vi "UHR-Fleezers Control (host) - 12.8.vi"() -> ()   [LabVIEW 2012] (continued)
                n1749 = Divide "X pix/step"(x=w2623, y=w2626) -> (x/y=w2632:dbl)
                n1750 = Negate(x=w2635) -> (-x=w2636:dbl)
                n1751 = local read "Initial Y"() -> (w2642:dbl)
                n1752 = Multiply(x=w2624, y=w2633) -> (x*y=w2643:dbl)
                n1753 = Divide "X half step offset"(x=w2621, y=2.0) -> (x/y=w2629:dbl)
                n1754 = Divide "X V/pix"(x=w2621, y=w2632) -> (x/y=w2631:dbl)
                n1755 = Multiply(x=w2621, y=w2626) -> (x*y=w2638:dbl)
                n1756 = Compound Arithmetic op=ADD(w2636, w2643, w2642) -> (w2613:dbl)
                "Pointer Y (V)" <- w2613
                n1757 = Multiply(x=w2631, y=w2625) -> (x*y=w2640:dbl)
                n1758 = Negate(x=w2629) -> (-x=w2628:dbl)
                n1759 = local read "Initial X"() -> (w2641:dbl)
                n1760 = Negate(x=w2640) -> (-x=w2639:dbl)
                n1761 = Compound Arithmetic op=ADD(w2628, w2638, w2641, w2639) -> (w2614:dbl)
                "Pointer X (V)" <- w2614
                n1762 = case shown="True" "Set High F Confocal Spot (X-Y)" {
                  tunnel: w2614 -> [_ w2644]
                  tunnel: w2613 -> [_ w2645]
                  frame False {
                  }
                  frame True {
                    "Confocal Y 2 (V)" <- w2645
                    "Confocal X 2 (V)" <- w2644
                  }
                }
                n1763 = Or(x="Set X Only", y="Set Confocal Spot (X-Y)") -> (x .or. y?=w2617:bool)
                n1764 = Or(x="Set Confocal Spot (X-Y)", y="Set Y Only") -> (x .or. y?=w2616:bool)
                n1765 = case shown="True" w2617 {
                  tunnel: w2614 -> [_ w2646]
                  frame False {
                  }
                  frame True {
                    n1766 = property on="AO2" class="Slide (strict)"("Val(Sgnl)"=w2646) -> ()  [unwired: 2 in, 2 out]
                    "Confocal X 1 (V)" <- w2646
                  }
                }
                n1767 = case shown="True" w2616 {
                  tunnel: w2613 -> [_ w2647]
                  frame False {
                  }
                  frame True {
                    n1768 = property on="AO1" class="Slide (strict)"("Val(Sgnl)"=w2647) -> ()  [unwired: 2 in, 2 out]
                    "Confocal Y 1 (V)" <- w2647
                  }
                }
                n1769 = local write "Set High F Confocal Spot (X-Y)"(w2612) -> ()
                n1770 = local write "Set Confocal Spot (X-Y)"(w2612) -> ()
                n1771 = local write "Set X Only"(w2612) -> ()
                n1772 = local write "Set Y Only"(w2612) -> ()
              }
            }
          }
          frame 3 {
            n1773 = local read "BD 2 Frequency 1 (MHz)"() -> (w2649:dbl)
            n1774 = local read "BD 1 Frequency 1 (MHz)"() -> (w2650:dbl)
            n1775 = local write "Manipulating Trap"(TRUE ("Manipulating Trap")) -> ()
            n1776 = local write "Coords"(T7 {"Horizontal"=0, "Vertical"=0} ("Coords")) -> ()
            n1777 = while {
              tunnel: w2654 -> [w2659]
              tunnel: w2652 -> [w2658]
              tunnel: w2650 -> [w2657]
              tunnel: w2649 -> [w2656]
              tunnel: w2648 -> [w2655]
              stop <- w2660 stop-if-true
              n1778 = event shown="[0] \"Pane\": Mouse Move" {
                selector: _ -> [_ _]
                dyn-events: _ -> [_ _]
                timeout: _ -> [_ _]
                tunnel: ["Force Manip Abort" w2724] -> w2660
                tunnel: w2659 -> [w2667 _]
                tunnel: w2658 -> [w2665 _]
                tunnel: w2657 -> [w2664 _]
                tunnel: w2656 -> [w2663 _]
                tunnel: w2655 -> [w2661 _]
                event Mouse Move {
                  n1779 = event-data() -> ("Time"=w2668:u32, "Coords"=w2669:T7)  [unwired: 3 out]
                  n1780 = Less?(x=w2668, y=w2667) -> (x < y?=w2666:bool)
                  n1781 = case "Makes sure old motion events prior to mouse click aren't used" shown="False" w2666 {
                    tunnel: w2669 -> [w2711 _]
                    tunnel: w2665 -> [w2712 _]
                    tunnel: w2664 -> [w2686 _]
                    tunnel: w2663 -> [w2685 _]
                    tunnel: w2661 -> [w2670 _]
                    frame False {
                      n1782 = Subtract(x=w2711, y=w2712) -> (x-y=w2710:T7)
                      "Coords" <- w2710
                      n1783 = local read "Y RF Frequency Limits (MHz)"() -> (w2671:T16)
                      n1784 = To Double Precision Float(number=w2710) -> (double precision float=w2709:cluster{"Horizontal":dbl, "Vertical":dbl})
                      n1785 = Multiply(x=cluster{"Horizontal":dbl, "Vertical":dbl} {"Horizontal"=-1.0, "Vertical"=1.0}, y="Manipulation Scaling") -> (x*y=w2705:cluster{"Horizontal":dbl, "Vertical":dbl})
                      n1786 = local read "X RF Frequency Limits (MHz)"() -> (w2672:T16)
                      n1787 = Multiply(x=w2709, y=w2705) -> (x*y=w2707:cluster{"Horizontal":dbl, "Vertical":dbl})
                      n1788 = Unbundle By Name(w2707) -> ("Horizontal"=w2702:dbl, "Vertical"=w2706:dbl)
                      n1789 = Unbundle By Name(w2671) -> ("Maximum"=w2674:dbl, "Minimum"=w2673:dbl)
                      n1790 = Boolean To (0,1)(Boolean="Manip. X?") -> (0, 1=w2700:i16)
                      n1791 = Boolean To (0,1)(Boolean="Manip. Y?") -> (0, 1=w2697:i16)
                      n1792 = local read "BD 1 Frequency 2 (MHz)"() -> (w2688:dbl)
                      n1793 = Multiply(x=w2706, y=w2697) -> (x*y=w2699:dbl)
                      n1794 = Multiply(x=w2700, y=w2702) -> (x*y=w2703:dbl)
                      n1795 = local read "BD 2 Frequency 2 (MHz)"() -> (w2687:dbl)
                      n1796 = Unbundle By Name(w2672) -> ("Maximum"=w2676:dbl, "Minimum"=w2675:dbl)
                      n1797 = Add(x=w2685, y=w2699) -> (x+y=w2678:dbl)
                      n1798 = Add(x=w2686, y=w2703) -> (x+y=w2680:dbl)
                      n1799 = In Range and Coerce(upper limit=w2676, x=w2680, lower limit=w2675) -> (coerced(x)=w2679:dbl)  [unwired: 1 out]
                      n1800 = In Range and Coerce(upper limit=w2674, x=w2678, lower limit=w2673) -> (coerced(x)=w2677:dbl)  [unwired: 1 out]
                      n1801 = Subtract(x=w2679, y=w2688) -> (x-y=w2696:dbl)
                      n1802 = Subtract(x=w2677, y=w2687) -> (x-y=w2695:dbl)
                      n1803 = Square(x=w2696) -> (x^2=w2694:dbl)
                      n1804 = Square(x=w2695) -> (x^2=w2693:dbl)
                      n1805 = Add(x=w2694, y=w2693) -> (x+y=w2692:dbl)
                      n1806 = Square Root(x=w2692) -> (sqrt(x)=w2689:dbl)
                      n1807 = In Range and Coerce(upper limit="Limit Max (MHz)", x=w2689, lower limit="Limit Min (MHz)") -> (In Range?=w2682:bool)  [unwired: 1 out]
                      n1808 = Not(x="Limits Enable") -> (.not. x?=w2681:bool)
                      n1809 = Or(x=w2682, y=w2681) -> (x .or. y?=w2683:bool)
                      n1810 = case shown="True" w2683 {
                        tunnel: w2689 -> [_ w2714]
                        tunnel: w2679 -> [_ w2721]
                        tunnel: w2688 -> [_ w2720]
                        tunnel: w2677 -> [_ w2719]
                        tunnel: w2687 -> [_ w2718]
                        tunnel: w2672 -> [_ w2716]
                        tunnel: w2671 -> [_ w2715]
                        tunnel: w2670 -> [_ w2713]
                        frame False {
                        }
                        frame True {
                          n1811 = local read "BD 1 Frequency 3 (MHz)"() -> (w2722:dbl)
                          n1812 = local read "BD 2 Frequency 3 (MHz)"() -> (w2717:dbl)
                          n1813 = local write "Trap Delta (MHz)"(w2714) -> ()
                          n1814 = call "set RF board frequency - interlace.vi"("Board 2 Frequency Limits"=w2715, "Board 1 Frequency Limits"=w2716, "FPGA VI Reference In"=w2713, "Board 2 Frequency 3 (MHz)"=w2717, "Board 1 Frequency 3 (MHz)"=w2722, "Board 2 Frequency 2 (MHz)"=w2718, "Board 2 Frequency 1 (MHz)"=w2719, "Board 1 Frequency 2 (MHz)"=w2720, "Board 1 Frequency 1  (MHz)"=w2721) -> ()  [unwired: 1 in, 2 out]
                          n1815 = local write "BD 2 Frequency 1 (MHz)"(w2719) -> ()
                          n1816 = local write "BD 1 Frequency 1 (MHz)"(w2721) -> ()
                        }
                      }
                    }
                    frame True {
                    }
                  }
                }
                event Mouse Up {
                  n1817 = event-data() -> ("Button"=w2723:u16)  [unwired: 8 out]
                  n1818 = case shown="3" w2723 {
                    tunnel: [FALSE TRUE] -> w2724
                    frame 0, Default {
                    }
                    frame 3 {
                      n1819 = local read "Trap Delta (MHz)"() -> (w2726:dbl)
                      n1820 = property on="Initial delta (MHz)" class="DigNum (strict)"("Val(Sgnl)"=w2726) -> ()  [unwired: 2 in, 2 out]
                      n1821 = local write "Manipulating Trap"(FALSE ("Manipulating Trap")) -> ()
                    }
                  }
                }
              }
            }
          }
        }
      }
      event Mouse Move {
        n1822 = event-data() -> ()  [unwired: 6 out]
      }
    }
    n1823 = local read "Stop All"() -> (w2542:bool)
    n1824 = node-c288() -> ()  [unwired: 2 out]
  }
  n1825 = flat-sequence "Video" {
    tunnel: [w2739] -> w55
    tunnel: w55 -> [w2780]
    frame #0 {
      w2729 = FALSE ("File open?")
      n1826 = while {
        stop <- w2731 continue-if-true
        n1827 = call "Close Video Capture.vi"() -> ("error code OUT"=w2733:i32)
        n1828 = Equal?(x=w2733, y=0) -> (x = y?=w2731:bool)
      }
      n1829 = local write "New Video File"(w2729) -> ()
      n1830 = local write "File open?"(w2729) -> ()
      n1831 = local write "Save Video"(w2729) -> ()
      n1832 = local write "Stop All"(FALSE ("Stop All")) -> ()
    }
    frame #1 {
      n1833 = call "DMR_Init.vi"() -> ()  [unwired: 3 out]
    }
    frame #2 {
      w2734 = "DE245428202"  # MSU fleezers card #
      (unwired) "DE019116701"  # Illinois fleezers card #
      # "Setting the destination format to Mono8 makes sure that the image can be displayed in the intensity plot."
      n1834 = call "DMR_GetDevice.vi"("search string IN"=w2734) -> ("device handle OUT"=w2757:i32)  [unwired: 4 in, 2 out]
      n1835 = call "DMR_OpenDevice.vi"("device handle IN"=w2757) -> ("driver handle OUT"=w2740:i32)  [unwired: 4 out]
      n1836 = call "DMR_FindList.vi"("flags IN"=u32 0 ("flags"), "list name IN"="" ("String"), "list type IN"=T35."camera descriptions", "driver handle IN"=w2740) -> ("list handle OUT"=w2743:i32)  [unwired: 2 out]
      n1837 = call "DMR_FindList.vi"("flags IN"=u32 0 ("flags"), "list name IN"="Base", "list type IN"=T35."setting", "driver handle IN"=w2740) -> ("list handle OUT"=w2741:i32)  [unwired: 2 out]
      n1838 = call "OBJ_GetHandle.vi"("object name IN"="VideoStandard", "list handle IN"=w2743) -> ("object handle OUT"=w2737:i32)  [unwired: 3 out]
      n1839 = call "OBJ_GetHandle.vi"("object name IN"="PixelFormat", "list handle IN"=w2741) -> ("object handle OUT"=w2751:i32)  [unwired: 3 out]
      n1840 = call "OBJ_SetS.vi"("value index IN"=0, "value IN"="NTSC M", "object handle IN"=w2737) -> ()  [unwired: 2 out]
      n1841 = call "OBJ_SetS.vi"("value index IN"=0, "value IN"="Mono8" ("value"), "object handle IN"=w2751) -> ()  [unwired: 2 out]
      n1842 = call "OBJ_GetHandle.vi"("object name IN"="VideoChannel", "list handle IN"=w2741) -> ("object handle OUT"=w2747:i32)  [unwired: 3 out]
      n1843 = while {
        tunnel: [w2761] -> w2739
        tunnel: w2740 -> [w2758]
        stop <- w2759 continue-if-true
        n1844 = call "DMR_ImageRequestSingle.vi"("request control IN"=0, "driver handle IN"=w2758) -> ("error code OUT"=w2760:i32, "driver handle OUT"=w2761:i32)  [unwired: 2 out]
        n1845 = Equal To 0?(x=w2760) -> (x = 0?=w2759:bool)
      }
      n1846 = call "OBJ_SetI.vi"("value index IN"=0, "value IN"=3 ("Video channel"), "object handle IN"=w2747) -> ()  [unwired: 2 out]
    }
    frame #3 {
      w2768 = T19 0 items=["Grayscale (U8)", "Grayscale (I16)", "Grayscale (SGL)", "Complex (CSG)", "RGB (U32)", "HSL (U32)", "RGB (U64)"] ("Image Type")
      w2776 = T19 0 items=["Grayscale (U8)", "Grayscale (I16)", "Grayscale (SGL)", "Complex (CSG)", "RGB (U32)", "HSL (U32)", "RGB (U64)"] ("Image Type")
      n1847 = call "IMAQ AVI2 Get Codec Names"() -> ("Codec Names"=w2763:string[])  [unwired: 10 in, 1 out]
      "Installed Codec Names" <- w2763
      n1848 = for "Create Greyscale map" {
        N: 256 -> [_]
        tunnel: [w2782] -> w2765 mode=indexing
        workers-P: _ -> [_]
        i -> [w2785]
        n1849 = To Unsigned Byte Integer(number=w2785) -> (unsigned 8bit integer=w2781:u8)
        n1850 = Join Numbers(hi=w2781, lo=w2781) -> ((hi.lo)=w2784:u16)
        n1851 = Join Numbers(hi=w2781, lo=w2781) -> ((hi.lo)=w2783:u16)
        n1852 = Join Numbers(hi=w2784, lo=w2783) -> ((hi.lo)=w2782:u32)
      }
      n1853 = property on="Codec choice" class="CmbBox"("Strings[]"=w2763) -> ()  [unwired: 2 in, 2 out]
      n1854 = call "IMAQ Create"("Image Name"="Scaled video", "Image Type"=w2768) -> ("New Image"=w2767:T2)  [unwired: 2 in, 2 out]
      n1855 = call "IMAQ Create"("Image Name"="Main video", "Image Type"=w2776) -> ("New Image"=w2777:T2)  [unwired: 2 in, 2 out]
      n1856 = node-c288(0 ("Processor")) -> (w2775:T23)  [unwired: 3 out]
      n1857 = Initialize Array(u32 0 ("Window Number (0...15)"), 480 ("dimension size"), 640 ("dimension size")) -> (w2770:u32[][])
      n1858 = timed-loop {
        tunnel: w2780 -> [w2802]
        tunnel: [w2801] -> w2779
        tunnel: w2777 -> [w2800]
        timing: w2775 -> [_]
        timing-out: [_] -> w2774
        tunnel: w2770 -> [w2793]
        tunnel: w2767 -> [w2791]
        tunnel: w2765 -> [w2790]
        stop <- w2792 stop-if-true
        # "This block performs the \nactual image capture."
        n1859 = node-c288() -> (→"Finished Late? [i-1]":bool)  [unwired: 5 out]
        n1860 = local read "Stop All"() -> (w2792:bool)
        n1861 = feedback #1(T36 refnum ("AVI Refnum")) -> (w2798:T36)
        n1862 = case shown="True" "New Video File" {
          tunnel: [w2815 w2816] -> w2789
          tunnel: w2798 -> [w2815 w2817]
          frame False {
          }
          frame True {
            n1863 = flat-sequence {
              tunnel: w2817 -> [w2819]
              tunnel: [w2821] -> w2816
              frame #0 {
                n1864 = local read "File open?"() -> (w2818:bool)
                n1865 = case shown="True" w2818 {
                  tunnel: w2819 -> [_ w2820]
                  frame False {
                  }
                  frame True {
                    n1866 = call "IMAQ AVI2 Close"("AVI Refnum"=w2820) -> ()  [unwired: 10 in, 1 out]
                  }
                }
              }
              frame #1 {
                n1867 = local write "New Video File"(FALSE ("New Video File")) -> ()
                n1868 = call "Create new save file.vi"("Ext"=".avi" ("string"), "Index In"="Video Index") -> ("Path Out"=w2824:path, "Index Out"=w2826:dbl)  [unwired: 1 in]
                "Path Out" <- w2824
                n1869 = local write "Video Index"(w2826) -> ()
                n1870 = call "IMAQ AVI2 Create"("Codec"="Codec choice", "Frames Per Second"=u32 30, "AVI Path"=w2824) -> ("AVI Refnum"=w2821:T36)  [unwired: 7 in, 1 out]
                "File open?" <- TRUE ("Files open?")
              }
            }
          }
        }
        n1871 = feedback-in #1(w2789) -> ()
        n1872 = call "DMR_ImageRequestWaitFor.vi"("queue number IN"=0, "timeout(ms) IN"=500, "driver handle IN"=w2802) -> ("error code OUT"=w2806:i32, "request number OUT"=w2803:i32, "driver handle OUT"=w2804:i32)
        n1873 = Equal To 0?(x=w2806) -> (x = 0?=w2805:bool)
        n1874 = Reciprocal(x="Video Capture Rate (Hz)") -> (1/x=w2796:dbl)
        n1875 = Multiply(x=w2796, y=1000.0) -> (x*y=w2794:dbl)
        n1876 = case shown="True" w2805 {
          tunnel: w2804 -> [w2830 w2867]
          tunnel: w2803 -> [_ w2866]
          tunnel: [w2830 w2863] -> w2801
          tunnel: w2800 -> [_ w2849]
          tunnel: w2793 -> [_ w2852]
          tunnel: w2789 -> [_ w2832]
          tunnel: w2791 -> [_ w2846]
          tunnel: w2790 -> [_ w2845]
          frame False {
          }
          frame True {
            w2857 = u32 0 ("X-offset IN")
            n1877 = call "DMR_GetImageRequestBufferData.vi"("driver handle IN"=w2867, "request number IN"=w2866) -> ("width OUT"=w2856:i32, "height OUT"=w2855:i32, "driver handle OUT"=w2862:i32, "request number OUT"=w2861:i32, "bytes per pixel OUT"=w2858:i32)  [unwired: 13 out]
            n1878 = call "DMR_GetImageRequestBufferImageData.vi"("driver handle IN"=w2862, "request number IN"=w2861, "bytes per pixel IN"=w2858, "X-offset IN"=w2857, "Y-offset IN"=w2857, "height IN"=w2855, "width IN"=w2856) -> ("driver handle OUT"=w2860:u32, "request number OUT"=w2859:u32, "image OUT"=w2838:u32[][])  [unwired: 10 out]
            n1879 = Transpose 2D Array(2D array=w2838) -> (transposed array=w2844:u32[][])
            n1880 = Select(t=w2844, s="Flip Y (or X)", f=w2838) -> (s? t:f=w2843:u32[][])
            n1881 = call "DMR_ImageRequestUnlock.vi"("request number IN"=w2859, "driver handle IN"=w2860) -> ("driver handle OUT"=w2865:i32)  [unwired: 1 in, 2 out]
            n1882 = for {
              tunnel: w2843 -> [w2902] mode=indexing
              tunnel: [w2901] -> w2841 mode=indexing
              n1883 = Reverse 1D Array(array=w2902) -> (reversed array=w2901:u32[])
            }
            n1884 = call "DMR_ImageRequestSingle.vi"("request control IN"=0, "driver handle IN"=w2865) -> ("driver handle OUT"=w2863:i32)  [unwired: 3 out]
            n1885 = Transpose 2D Array(2D array=w2841) -> (transposed array=w2842:u32[][])
            n1886 = Select(t=w2842, s="Flip Y (or X)", f=w2841) -> (s? t:f=w2839:u32[][])
            n1887 = Select(t=w2839, s="Flip Image", f=w2838) -> (s? t:f=w2836:u32[][])
            n1888 = case shown="True" "Averaging" {
              tunnel: w2836 -> [w2913 w2918]
              tunnel: [w2913 w2917] -> w2850
              tunnel: w2852 -> [_ w2915]
              frame False {
              }
              frame True {
                (unwired) 1
                w2923 = 1
                n1889 = feedback #2(w2915) -> (w2914:u32[][])
                n1890 = Add(x=w2918, y=w2914) -> (x+y=w2919:u32[][])
                n1891 = Select(t=w2915, s="Reset Averaging", f=w2919) -> (s? t:f=w2921:u32[][])
                n1892 = feedback-in #2(w2921) -> ()
                n1893 = feedback #3(w2923) -> (w2916:i32)
                n1894 = Divide(x=w2919, y=w2916) -> (x/y=w2920:dbl[][])
                n1895 = Increment(x=w2916) -> (x+1=w2924:i32)
                n1896 = To Unsigned Long Integer(number=w2920) -> (unsigned 32bit integer=w2917:u32[][])
                n1897 = Select(t=w2923, s="Reset Averaging", f=w2924) -> (s? t:f=w2922:i32)
                n1898 = feedback-in #3(w2922) -> ()
              }
            }
            n1899 = case shown="True" "Zoom video window" {
              tunnel: w2850 -> [_ w2881]
              tunnel: w2846 -> [_ w2880]
              frame False {
              }
              frame True {
                n1900 = To Double Precision Float(number=w2881) -> (double precision float=w2878:dbl[][])
                n1901 = In Range and Coerce(upper limit="Intensity Upper", x=w2878, lower limit="Intensity Lower") -> (coerced(x)=w2877:dbl[][])  [unwired: 1 out]
                n1902 = Subtract(x="Intensity Upper", y="Intensity Lower") -> (x-y=w2874:dbl)
                n1903 = Subtract(x=w2877, y="Intensity Lower") -> (x-y=w2875:dbl[][])
                n1904 = Divide(x=w2875, y=w2874) -> (x/y=w2876:dbl[][])
                n1905 = Multiply(x=255.0, y=w2876) -> (x*y=w2872:dbl[][])
                n1906 = To Unsigned Byte Integer(number=w2872) -> (unsigned 8bit integer=w2879:u8[][])
                n1907 = call "IMAQ ArrayToImage"("Image Pixels (U8)"=w2879, "Image"=w2880) -> ("Image Out"=w2868:T2)  [unwired: 4 in, 5 out]
                n1908 = First Call?() -> (First Call?: T/F=w2869:bool)
                n1909 = case shown="True" w2869 {
                  tunnel: w2868 -> [w2882 w2893]
                  frame False {
                    n1910 = flat-sequence {
                      tunnel: w2882 -> [w2888]
                      frame #0 {
                        w2885 = FALSE ("Get/Set Status? (Set)")
                        w2884 = 0 ("Window Number (0...15)")
                        n1911 = call "IMAQ WindSize"("Get/Set Status? (Set)"=w2885, "Window Number"=w2884) -> ("Width & Height out"=→"Window Size":cluster{"Width":i32, "Height":i32})  [unwired: 4 in, 2 out]
                        n1912 = call "IMAQ WindMove"("Window Number (0...15)"=w2884, "Get/Set Status? (Set)"=w2885) -> ("Coordinates (screen)"=→"Window Position":cluster{"X Position":i32, "Y Position":i32})  [unwired: 3 in, 1 out]
                        n1913 = call "IMAQ WindDraw"("Resize to Image Size? (Y)"=FALSE, "Window Number (0...15)"=w2884, "Image"=w2888) -> ()  [unwired: 7 in, 2 out]
                      }
                      frame #1 {
                        n1914 = call "IMAQ WindZoom 2"("Center Point"="Center Point", "Zoom to Fit? (False)"=FALSE, "Zoom Factor"="Zoom Factor") -> ()  [unwired: 5 in, 4 out]
                      }
                    }
                  }
                  frame True {
                    n1915 = flat-sequence {
                      tunnel: w2893 -> [w2896]
                      tunnel: [w2894] -> w2892
                      tunnel: w2892 -> [w2898]
                      frame #0 {
                        w2895 = TRUE ("Resize to Image Size? (Y)")
                        w2894 = 0 ("Window Number (0...15)")
                        n1916 = call "IMAQ WindNonTearing"("Window Number"=w2894, "NonTearing? (True)"=w2895) -> ()  [unwired: 8 in, 2 out]
                        n1917 = call "IMAQ WindDraw"("Resize to Image Size? (Y)"=w2895, "Window Number (0...15)"=w2894, "Image"=w2896) -> ()  [unwired: 7 in, 2 out]
                      }
                      frame #1 {
                        n1918 = call "IMAQ WindSize"("Scrollbars? (N)"=FALSE, "Width & Height"="Initial Window Size", "Window Number"=w2898) -> ()  [unwired: 3 in, 3 out]
                        n1919 = call "IMAQ WindMove"("Window Number (0...15)"=w2898, "Coordinates (screen)"="Initial Window Position") -> ()  [unwired: 3 in, 2 out]
                      }
                    }
                  }
                }
              }
            }
            n1920 = To Unsigned Byte Integer(number=w2850) -> (unsigned 8bit integer=w2848:u8[][])
            n1921 = call "IMAQ ArrayToImage"("Image Pixels (U8)"=w2848, "Image"=w2849) -> ("Image Out"=w2847:T2)  [unwired: 4 in, 5 out]
            "Primary Video Display" <- w2847
            n1922 = Not(x="Close Video File") -> (.not. x?=w2834:bool)
            n1923 = And(x="Save Video", y=w2834) -> (x .and. y?=w2831:bool)
            n1924 = case shown="True" "Save Image" {
              tunnel: w2848 -> [_ w2927]
              tunnel: w2845 -> [_ w2926]
              frame False {
              }
              frame True {
                n1925 = call <vilib>:"Flatten Pixmap.vi"("colors"=w2926, "8-bit pixmap"=w2927) -> ("image data"=w2933:T37)  [unwired: 4 in, 5 out]
                n1926 = call "Create new save file.vi"("Insert"="video_frame_" ("string"), "Ext"=".bmp" ("string"), "Index In"="Image Index") -> ("Path Out"=w2929:path, "Index Out"=w2934:dbl)
                n1927 = Increment(x=w2934) -> (x+1=w2928:dbl)
                n1928 = local write "Image Index"(w2928) -> ()
                n1929 = call <vilib>:"Write BMP File.vi"("image data"=w2933, "path to BMP file"=w2929) -> ()  [unwired: 1 in, 9 out]
              }
            }
            n1930 = case shown="True" w2831 {
              tunnel: w2832 -> [w2904 w2909]
              tunnel: w2847 -> [_ w2908]
              tunnel: "Close Video File" -> [w2903 _]
              frame False {
                n1931 = case shown="True" w2903 {
                  tunnel: w2904 -> [_ w2905]
                  frame False {
                  }
                  frame True {
                    w2906 = FALSE ("Save Video")
                    n1932 = call "IMAQ AVI2 Close"("AVI Refnum"=w2905) -> ()  [unwired: 10 in, 1 out]
                    n1933 = local write "File open?"(w2906) -> ()
                    n1934 = local write "Save Video"(w2906) -> ()
                  }
                }
              }
              frame True {
                n1935 = local read "File open?"() -> (w2907:bool)
                n1936 = case shown="True" w2907 {
                  tunnel: w2909 -> [_ w2912]
                  tunnel: w2908 -> [_ w2911]
                  frame False {
                    n1937 = local write "New Video File"(TRUE ("New Video File")) -> ()
                  }
                  frame True {
                    n1938 = call "IMAQ AVI2 Write Frame"("Image"=w2911, "AVI Refnum"=w2912) -> ()  [unwired: 7 in, 3 out]
                  }
                }
              }
            }
          }
        }
        n1939 = node-c288(w2794, "Deadline (ms)") -> ()  [unwired: 1 out]
      }
      n1940 = node-c288(w2774) -> ()  [unwired: 1 out]
      n1941 = call "DMR_CloseDevice.vi"("driver handle IN"=w2779) -> ()  [unwired: 1 in, 4 out]
    }
    frame #4 {
      n1942 = call "DMR_Close.vi"() -> ()  [unwired: 1 out]
    }
  }
  n1943 = node-c288(3 ("Processor")) -> (w64:T23)  [unwired: 3 out]
  n1944 = timed-loop "Oscillate Trap/AOM (fishing, conjugate plane alignment)" {
    tunnel: [w2940] -> w69
    timing: w64 -> [_]
    timing-out: [_] -> w63
    tunnel: w5 -> [w2939]
    stop <- w2940 stop-if-true
    n1945 = node-c288() -> ()  [unwired: 2 out]
    n1946 = event shown="[0] \"Oscillate Set 1\", \"Fish for Tether\": Value Change" {
      selector: _ -> [_ _ _]
      dyn-events: _ -> [_ _ _]
      timeout: _ -> [_ _ _]
      tunnel: [FALSE ("Stop All") _ w3545] -> w2940
      tunnel: w2939 -> [w2943 _ _]
      event "Oscillate Set 1", "Fish for Tether": Value Change {
        n1947 = event-data() -> ()  [unwired: 6 out]
        n1948 = local read "Oscillate Set 1"() -> (w2947:bool)
        n1949 = Or(x=w2947, y="Fish for Tether") -> (x .or. y?=w2945:bool)
        n1950 = case shown="True" w2945 {
          tunnel: "Fish for Tether" -> [_ w2950]
          tunnel: w2943 -> [_ w2948]
          frame False {
          }
          frame True {
            n1951 = case shown="True" w2950 {
              selector: w2950 -> [w2953 w2959]
              tunnel: [w2953 w2959] -> w2949
              frame False {
              }
              frame True {
                n1952 = local write "Scan axis 2"(TRUE) -> ()
                n1953 = local write "Tether"(FALSE ("Tether")) -> ()
                n1954 = local read "Flow ON during cal?"() -> (w2954:bool)
                n1955 = property on="Trap Delta (MHz)" class="DigNum (strict)"("Val(Sgnl)"="Furthest Delta (MHz)") -> ()  [unwired: 2 in, 2 out]
                n1956 = Or(x="Flow ON during \nfishing?", y=w2954) -> (x .or. y?=w2955:bool)
                n1957 = Wait (ms)(milliseconds to wait=u32 500) -> ()  [unwired: 1 out]
                n1958 = property on="Sample Channel\nFlow" class="Bool (strict)"("Val(Sgnl)"=w2955) -> ()  [unwired: 2 in, 2 out]
              }
            }
            n1959 = node-c288() -> (w2952:T23)  [unwired: 1 in, 3 out]
            n1960 = timed-loop "Oscillate AOD" {
              timing: w2952 -> [_]
              timing-out: [_] -> w2951
              tunnel: w2949 -> [w2963]
              tunnel: w2948 -> [w2962]
              i -> [w2971]
              stop <- w2969 stop-if-true
              n1961 = node-c288() -> (w2970:i64)  [unwired: 1 out]
              n1962 = flat-sequence {
                tunnel: w2971 -> [w2998]
                tunnel: w2970 -> [w2997]
                tunnel: w2963 -> [w2981]
                tunnel: [w2981] -> w2968
                tunnel: [w2980] -> w2967
                tunnel: [w2979] -> w2966
                tunnel: [w2976] -> w2964
                tunnel: w2962 -> [w2972]
                tunnel: w2968 -> [w3043]
                tunnel: w2967 -> [w3041]
                tunnel: w2966 -> [w3040]
                tunnel: [w3039] -> w2965
                tunnel: w2964 -> [w3038]
                tunnel: [w3115] -> w2969
                tunnel: w2965 -> [w3114]
                frame #0 {
                  # "w (rad/s)"
                  # "t (s)"
                  n1963 = Divide(x=w2997, y=i64 1000) -> (x/y=w2973:dbl)
                  n1964 = local read "BD 1 Frequency 2 (MHz)"() -> (w2975:dbl)
                  n1965 = Multiply(x="Osc. freq. (Hz)", y=6.283185307179586) -> (x*y=w2995:dbl)
                  n1966 = Multiply(x=w2973, y=w2998) -> (x*y=w2994:dbl)
                  n1967 = Multiply(x=w2995, y=w2994) -> (x*y=w2978:dbl)
                  n1968 = local read "BD 1 Frequency 1 (MHz)"() -> (w2983:dbl)
                  n1969 = case shown="True" w2981 {
                    tunnel: w2978 -> [w3004 w3021]
                    tunnel: w2983 -> [_ w3029]
                    tunnel: w2975 -> [_ w3030]
                    tunnel: [w3001 w3025] -> w2974
                    tunnel: [FALSE w3006] -> w2979
                    tunnel: [0.0 w3017] -> w2976
                    frame False {
                      n1970 = Sine(x=w3004) -> (sin(x)=w3002:dbl)
                      n1971 = Multiply(x=w3002, y="Osc. amp. (MHz)") -> (x*y=w3001:dbl)
                    }
                    frame True {
                      # "trap position goes from 0 to 1 (0 is when it is furthest away, 1 is when closest)\nso we want to test for tether only when farther away, or x < 1"
                      # "quit if taking too long"
                      # "oscillate the trap"
                      # "Test for tether"
                      n1972 = local read "Vec Mean of T1 T2"() -> (w3005:dbl[])
                      "Trigger Signal" <- w3005
                      n1973 = Cosine(x=w3021) -> (cos(x)=w3033:dbl)
                      n1974 = Subtract(x=w3030, y=w3029) -> (x-y=w3028:dbl)
                      n1975 = Decrement(x=w3033) -> (x-1=w3032:dbl)
                      n1976 = Subtract(x=w3028, y="Closest Delta (MHz)") -> (x-y=w3026:dbl)
                      n1977 = Divide(x=w3032, y=-2.0) -> (x/y=w3016:dbl)
                      n1978 = Greater?(x=w3005, y="Stop F (pN)") -> (0:w3023:bool[])
                      n1979 = Multiply(x=w3016, y=w3026) -> (x*y=w3025:dbl)
                      n1980 = Less?(x=w3016, y="Fish mask thresh") -> (x < y?=w3015:bool)
                      n1981 = Boolean To (0,1)(Boolean=w3015) -> (0, 1=w3013:i16)
                      n1982 = Multiply(x=w3013, y=w3005) -> (x*y=w3012:dbl[])
                      n1983 = Divide(x=w3021, y=6.283185307179586) -> (x/y=w3020:dbl)
                      n1984 = Round Toward +Infinity(x=w3020) -> (ceil(x): smallest int >= x=w3017:dbl)
                      "Attempts" <- w3017
                      n1985 = Greater?(x=w3012, y="Stop F (pN) (mask)") -> (0:w3010:bool[])
                      n1986 = Or Array Elements(Boolean array=w3023) -> (logical OR=w3008:bool)
                      n1987 = Or Array Elements(Boolean array=w3010) -> (logical OR=w3007:bool)
                      n1988 = Greater?(x=w3017, y="Attempt Limit") -> (0:w3019:bool)
                      n1989 = case shown="True" w3019 {
                        frame False {
                        }
                        frame True {
                          n1990 = local write "Fish for Tether"(FALSE ("Fish for Tether")) -> ()
                          n1991 = call <vilib>:"Beep.vi"() -> ()  [unwired: 3 in, 9 out]
                          n1992 = local read "Messages"() -> (w3035:string)
                          n1993 = call "Update messages.vi"("Message to add"="Tether fishing timeout." ("Messages"), "Old message string"=w3035) -> ("New message string"=→"Messages":string)
                        }
                      }
                      n1994 = Select(t=w3008, s="Normal (on) or masked test (off)", f=w3007) -> (s? t:f=w3006:bool)
                    }
                  }
                  n1995 = local read "BD 2 Frequency 1 (MHz)"() -> (w2982:dbl)
                  n1996 = Select(t=w2983, s="Scan axis 2", f=w2982) -> (s? t:f=w2986:dbl)
                  n1997 = Add(x=w2974, y=w2986) -> (x+y=w2980:dbl)
                  n1998 = Select(t=w2980, s="Scan axis 2", f=w2983) -> (s? t:f=w2989:dbl)
                  n1999 = Select(t=w2982, s="Scan axis 2", f=w2980) -> (s? t:f=w2988:dbl)
                  n2000 = local read "BD 2 Frequency 2 (MHz)"() -> (w2991:dbl)
                  n2001 = local read "BD 2 Frequency 3 (MHz)"() -> (w2990:dbl)
                  n2002 = local read "Y RF Frequency Limits (MHz)"() -> (w2984:T16)
                  n2003 = local read "X RF Frequency Limits (MHz)"() -> (w2985:T16)
                  n2004 = local read "BD 1 Frequency 3 (MHz)"() -> (w2992:dbl)
                  n2005 = call "set RF board frequency - interlace.vi"("Board 2 Frequency Limits"=w2984, "Board 1 Frequency Limits"=w2985, "FPGA VI Reference In"=w2972, "Board 2 Frequency 3 (MHz)"=w2990, "Board 1 Frequency 3 (MHz)"=w2992, "Board 2 Frequency 2 (MHz)"=w2991, "Board 2 Frequency 1 (MHz)"=w2988, "Board 1 Frequency 2 (MHz)"=w2975, "Board 1 Frequency 1  (MHz)"=w2989) -> ()  [unwired: 1 in, 2 out]
                }
                frame #1 {
                  n2006 = And(x=w3043, y=w3040) -> (x .and. y?=w3042:bool)
                  n2007 = case "Only if were fishing and now formed tether" shown="True" w3042 {
                    tunnel: w3041 -> [w3045 w3060]
                    tunnel: [w3044 w3059] -> w3039
                    tunnel: w3038 -> [_ w3055]
                    frame False {
                      n2008 = local read "Fish for Tether"() -> (w3044:bool)
                      n2009 = case shown="False" w3044 {
                        tunnel: w3045 -> [w3046 _]
                        frame False {
                          n2010 = property on="BD 1 Frequency 1 (MHz)" class="DigNum (strict)"("Val(Sgnl)"=w3046) -> ()  [unwired: 2 in, 2 out]
                        }
                        frame True {
                        }
                      }
                    }
                    frame True {
                      w3059 = FALSE ("Fish for Tether")
                      n2011 = call <vilib>:"Beep.vi"() -> ()  [unwired: 3 in, 9 out]
                      n2012 = Number To Decimal String(number=w3055, width (-)=i16 1) -> (decimal integer string=w3053:string)
                      n2013 = Concatenate Strings("Formed tether in ", w3053, " attempt(s)." ("string")) -> (w3050:string)
                      n2014 = local read "Messages"() -> (w3057:string)
                      n2015 = local write "Fish for Tether"(w3059) -> ()
                      n2016 = call "Update messages.vi"("Message to add"=w3050, "Old message string"=w3057) -> ("New message string"=w3056:string)
                      n2017 = local write "Messages"(w3056) -> ()
                      n2018 = Get Date/Time In Seconds() -> (seconds since 1Jan1904=→"Time tether formed":timestamp)
                      n2019 = local read "Flow ON during cal?"() -> (w3047:bool)
                      n2020 = property on="Sample Channel\nFlow" class="Bool (strict)"("Val(Sgnl)"=w3047) -> (error out=w3048:errorcluster)  [unwired: 2 in, 1 out]
                      n2021 = case shown="\"2\", \"3\", \"4\", \"5\", \"6\"" "Then..." {
                        selector: "Then..." -> [_ w3063]
                        tunnel: w3060 -> [w3062 _]
                        tunnel: w3048 -> [_ _]
                        frame "1", Default {
                          n2022 = property on="BD 1 Frequency 1 (MHz)" class="DigNum (strict)"("Val(Sgnl)"=w3062) -> ()  [unwired: 2 in, 2 out]
                        }
                        frame "2", "3", "4", "5", "6" {
                          n2023 = flat-sequence {
                            tunnel: w3063 -> [w3065]
                            frame #0 {
                              n2024 = property on="Trap Delta (MHz)" class="DigNum (strict)"("Val(Sgnl)"="Move to Delta 1 (MHz)") -> ()  [unwired: 2 in, 2 out]
                            }
                            frame #1 {
                              n2025 = case shown="\"5\", \"6\"" w3065 {
                                selector: w3065 -> [w3068 w3078 _]
                                frame "3", "4" {
                                n2026 = flat-sequence {
                                tunnel: w3068 -> [w3069]
                                tunnel: [w3069] -> w3066
                                tunnel: [w3071] -> w3067
                                tunnel: w3066 -> [w3071]
                                tunnel: w3067 -> [w3075]
                                frame #0 {
                                n2027 = property on="Green Laser ON" class="Bool (strict)"("Val(Sgnl)"=TRUE ("Value (Signaling)")) -> ()  [unwired: 2 in, 2 out]
                                }
                                frame #1 {
                                n2028 = Multiply(x="Wait Before Save (s)", y=u32 1000 ("x")) -> (x*y=w3073:u32)
                                n2029 = Wait (ms)(milliseconds to wait=w3073) -> ()  [unwired: 1 out]
                                }
                                frame #2 {
                                n2030 = property on="Start Saving" class="Bool (strict)"("Value"=TRUE ("Start Saving")) -> ()  [unwired: 2 in, 2 out]
                                n2031 = case shown="\"4\"" w3075 {
                                frame Default {
                                }
                                frame "4" {
                                n2032 = property on="Fl. Triggered..." class="Bool (strict)"("Val(Sgnl)"=TRUE ("Value (Signaling)")) -> ()  [unwired: 2 in, 2 out]
                                }
                                }
                                }
                                }
                                }
                                frame "5", "6" {
                                n2033 = stacked-sequence {
                                tunnel: w3078 -> [_ _ _ _ _ _ w3090]
                                frame #0 {
                                n2034 = Replace Array Subset(array=u32[] [0] ("Index Values"), new element="Raster Set Upon Tether", index=0) -> (w3079:u32[])
                                n2035 = property on="Saved AOD Raster Scan Parameter Sets" class="Arr (strict)"("Index Values"=w3079) -> ()  [unwired: 2 in, 2 out]
                                }
                                frame #1 {
                                n2036 = Wait (ms)(milliseconds to wait=u32 500) -> ()  [unwired: 1 out]
                                }
                                frame #2 {
                                n2037 = property on="Load parameters" class="Bool (strict)"("Val(Sgnl)"=TRUE ("Value (Signaling)")) -> ()  [unwired: 2 in, 2 out]
                                n2038 = case shown="True" "Green ON During Raster" {
                                frame False {
                                }
                                frame True {
                                n2039 = property on="Green Laser ON" class="Bool (strict)"("Val(Sgnl)"=TRUE ("Value (Signaling)")) -> ()  [unwired: 2 in, 2 out]
                                }
                                }
                                }
                                frame #3 {
                                n2040 = Wait (ms)(milliseconds to wait=u32 500) -> ()  [unwired: 1 out]
                                }
                                frame #4 {
                                n2041 = property on="Trap Raster Scan" class="Bool (strict)"("Val(Sgnl)"=TRUE ("Value (Signaling)")) -> ()  [unwired: 2 in, 2 out]
                                }
                                frame #5 {
                                n2042 = Wait (ms)(milliseconds to wait=u32 2000) -> ()  [unwired: 1 out]
                                }
                                frame #6 {
                                n2043 = flat-sequence {
                                tunnel: w3090 -> [w3097]
                                frame #0 {
                                n2044 = while {
                                stop <- w3093 stop-if-true
                                n2045 = local read "Raster Scanning..."() -> (w3092:bool)
                                n2046 = local read "Saving..."() -> (w3095:bool)
                                n2047 = Wait (ms)(milliseconds to wait=u32 100) -> ()  [unwired: 1 out]
                                n2048 = Not(x=w3095) -> (.not. x?=w3094:bool)
                                n2049 = Not(x=w3092) -> (.not. x?=w3091:bool)
                                n2050 = And(x=w3094, y=w3091) -> (x .and. y?=w3093:bool)
                                }
                                }
                                frame #1 {
                                n2051 = local read "Tether"() -> (w3098:bool)
                                n2052 = case shown="True" w3098 {
                                tunnel: w3097 -> [_ w3100]
                                frame False {
                                n2053 = property on="Fish for Tether" class="Bool (strict)"("Val(Sgnl)"="Fish again after \nraster break?") -> ()  [unwired: 2 in, 2 out]
                                }
                                frame True {
                                n2054 = stacked-sequence {
                                tunnel: w3100 -> [_ w3104 _ _]
                                frame #0 {
                                n2055 = property on="Trap Delta (MHz)" class="DigNum (strict)"("Val(Sgnl)"="Move to Delta 2 (MHz)") -> ()  [unwired: 2 in, 2 out]
                                n2056 = case shown="True" "Flow ON after\ntether testing?" {
                                frame False {
                                }
                                frame True {
                                n2057 = property on="Sample Channel\nFlow" class="Bool (strict)"("Val(Sgnl)"=TRUE ("Value (Signaling)")) -> ()  [unwired: 2 in, 2 out]
                                }
                                }
                                }
                                frame #1 {
                                n2058 = flat-sequence {
                                tunnel: w3104 -> [w3106]
                                frame #0 {
                                n2059 = Wait (ms)(milliseconds to wait=u32 500) -> ()  [unwired: 1 out]
                                }
                                frame #1 {
                                n2060 = case shown="\"6\"" w3106 {
                                frame Default {
                                }
                                frame "6" {
                                n2061 = property on="Green Laser ON" class="Bool (strict)"("Val(Sgnl)"=TRUE ("Green Laser ON/Interlacing")) -> ()  [unwired: 2 in, 2 out]
                                }
                                }
                                }
                                frame #2 {
                                n2062 = Wait (ms)(milliseconds to wait=u32 500) -> ()  [unwired: 1 out]
                                }
                                frame #3 {
                                n2063 = local write "Start Saving"("Save at end (5, 6)") -> ()
                                }
                                }
                                }
                                frame #2 {
                                n2064 = local read "Bead Sep. Int. Time (s)"() -> (w3112:dbl)
                                n2065 = Multiply(x=w3112, y=1000.0) -> (x*y=w3111:dbl)
                                n2066 = Wait (ms)(milliseconds to wait=w3111) -> ()  [unwired: 1 out]
                                }
                                frame #3 {
                                n2067 = property on="Remove Offset" class="Bool (strict)"("Val(Sgnl)"=TRUE ("Value (Signaling)")) -> ()  [unwired: 2 in, 2 out]
                                }
                                }
                                }
                                }
                                }
                                }
                                }
                                }
                                }
                                frame "2", Default {
                                }
                              }
                            }
                          }
                        }
                      }
                      "Tether" <- "Tether Alarm?"
                    }
                  }
                }
                frame #2 {
                  n2068 = local read "Oscillate Set 1"() -> (w3119:bool)
                  n2069 = local read "Stop All"() -> (w3117:bool)
                  n2070 = Or(x=w3119, y=w3114) -> (x .or. y?=w3116:bool)
                  n2071 = Not(x=w3116) -> (.not. x?=w3118:bool)
                  n2072 = Compound Arithmetic op=OR(w3117, w3118) -> (w3115:bool)
                }
              }
              n2073 = node-c288() -> ()  [unwired: 2 out]
            }
            n2074 = node-c288(w2951) -> ()  [unwired: 1 out]
          }
        }
      }
      event "Fl. Triggered...": Value Change {
        n2075 = event-data() -> ()  [unwired: 7 out]
        n2076 = case shown="True" "Fl. Triggered..." {
          frame False {
          }
          frame True {
            n2077 = node-c288() -> (w3130:T23)  [unwired: 4 out]
            n2078 = timed-loop {
              timing: w3130 -> [_]
              timing-out: [_] -> w3129
              tunnel: "Action" -> [w3138]
              shift-right: [w3135] -> _
              shift-left: u8 255 -> [w3137]
              shift-right: [w3132] -> _
              shift-left: 255 -> [w3134]
              stop <- w3131 stop-if-true
              # "Reset confocal spot"
              n2079 = node-c288() -> ()  [unwired: 2 out]
              n2080 = flat-sequence {
                tunnel: w3138 -> [w3158]
                tunnel: w3137 -> [w3157]
                tunnel: [w3156] -> w3136
                tunnel: w3134 -> [w3143]
                tunnel: [w3142] -> w3133
                tunnel: [w3537] -> w3131
                tunnel: w3136 -> [w3536]
                tunnel: [w3536] -> w3135
                tunnel: [w3535] -> w3132
                tunnel: w3133 -> [w3535]
                frame #0 {
                  n2081 = local read "Delta Fl. 2"() -> (w3155:dbl)
                  n2082 = local read "Delta Fl. 1"() -> (w3150:dbl)
                  n2083 = Multiply(x="Fl. Delta Thresh. (kHz)", y=1000.0) -> (x*y=w3145:dbl)
                  n2084 = Select(t=w3150, s="APD to Watch", f=w3155) -> (s? t:f=w3146:dbl)
                  n2085 = Greater?(x=w3146, y=w3145) -> (0:w3151:bool)
                  n2086 = Or(x="Force Yank", y=w3151) -> (x .or. y?=w3149:bool)
                  n2087 = And(x=w3149, y="Yank when?") -> (x .and. y?=w3147:bool)
                  n2088 = case shown="False" w3147 {
                    tunnel: w3158 -> [w3161 w3362]
                    tunnel: w3157 -> [w3163 w3358]
                    tunnel: [w3163 w3356] -> w3156
                    tunnel: w3146 -> [w3169 _]
                    tunnel: w3145 -> [w3168 _]
                    tunnel: "Force Yank" -> [w3166 _]
                    tunnel: w3143 -> [w3165 w3355]
                    tunnel: [w3164 w3355] -> w3142
                    frame False {
                      n2089 = Negate(x=w3168) -> (-x=w3160:dbl)
                      n2090 = local write "Fl. High"(TRUE ("Fl. High")) -> ()
                      n2091 = Less?(x=w3169, y=w3160) -> (x < y?=w3167:bool)
                      n2092 = Or(x=w3166, y=w3167) -> (x .or. y?=w3162:bool)
                      n2093 = case shown="True" w3162 {
                        tunnel: w3165 -> [w3170 w3180]
                        tunnel: [w3170 w3179] -> w3164
                        tunnel: w3161 -> [_ w3178]
                        frame False {
                        }
                        frame True {
                          n2094 = flat-sequence {
                            tunnel: w3180 -> [w3186]
                            tunnel: w3178 -> [w3183]
                            tunnel: [w3185] -> w3177
                            tunnel: [w3184] -> w3176
                            tunnel: [w3183] -> w3175
                            tunnel: w3174 -> [w3182]
                            tunnel: [w3182] -> w3173
                            tunnel: w3172 -> [w3181]
                            tunnel: [w3181] -> w3171
                            tunnel: [w3257] -> w3179
                            tunnel: w3177 -> [w3257]
                            tunnel: w3176 -> [w3256]
                            tunnel: w3175 -> [w3255]
                            tunnel: w3173 -> [w3254]
                            tunnel: w3171 -> [w3253]
                            frame #0 {
                              n2095 = call <vilib>:"Beep.vi"() -> ()  [unwired: 12 in]
                              n2096 = local write "Waiting"(FALSE ("Waiting")) -> ()
                              n2097 = Increment(x=w3186) -> (x+1=w3185:i32)
                              n2098 = case shown="\"Image\"" w3183 {
                                tunnel: w3185 -> [_ w3191 _]
                                frame "Alarm", Default {
                                }
                                frame "Yank" {
                                n2099 = flat-sequence {
                                tunnel: w3191 -> [w3194]
                                tunnel: [w3193] -> w3190
                                tunnel: [w3192] -> w3189
                                tunnel: w3190 -> [w3204]
                                tunnel: w3189 -> [w3205]
                                frame #0 {
                                n2100 = local read "Yank Delay (s)"() -> (w3197:dbl)
                                n2101 = local read "N Array El"() -> (w3192:u8)
                                n2102 = Quotient & Remainder(x=w3194, y=w3192) -> (x-y*floor(x/y)=w3193:i32)  [unwired: 1 out]
                                n2103 = Multiply(x=w3197, y=1000.0) -> (x*y=w3195:dbl)
                                n2104 = Wait (ms)(milliseconds to wait=w3195) -> ()  [unwired: 1 out]
                                }
                                frame #1 {
                                n2105 = local read "Yank to which?"() -> (w3199:bool)
                                n2106 = local read "Random Choice"() -> (w3209:bool)
                                n2107 = local read "Yank to Trap Delta (MHz)"() -> (w3202:dbl[])
                                n2108 = local read "Yank to SP"() -> (w3203:dbl[])
                                n2109 = Random Number (0-1)() -> (number: 0 to 1=w3208:dbl)
                                n2110 = Multiply(x=w3205, y=w3208) -> (x*y=w3207:dbl)
                                n2111 = Round Toward -Infinity(1:w3207) -> (0:w3206:dbl)
                                n2112 = Select(t=w3206, s=w3209, f=w3204) -> (s? t:f=w3200:dbl)
                                n2113 = Select(t=w3202, s=w3199, f=w3203) -> (s? t:f=w3201:dbl[])
                                n2114 = Index Array(array=w3201, index=w3200) -> (element=w3198:dbl)
                                n2115 = case shown="True" w3199 {
                                tunnel: w3198 -> [w3210 w3237]
                                frame False {
                                n2116 = flat-sequence {
                                tunnel: w3210 -> [w3211]
                                frame #0 {
                                n2117 = property on="Trap Pos FB SP" class="DigNum (strict)"("Val(Sgnl)"=w3211) -> ()  [unwired: 2 in, 2 out]
                                }
                                frame #1 {
                                n2118 = Wait (ms)(milliseconds to wait=u32 700) -> ()  [unwired: 1 out]
                                }
                                frame #2 {
                                n2119 = local read "Action (%)"() -> (w3216:dbl)
                                n2120 = Absolute Value(x=w3216) -> (abs(x)=w3215:dbl)
                                n2121 = Greater?(x=w3215, y=70.0) -> (0:w3213:bool)
                                n2122 = property on="Remove Action Offset" class="Bool (strict)"("Val(Sgnl)"=w3213) -> ()  [unwired: 2 in, 2 out]
                                }
                                frame #3 {
                                n2123 = for {
                                N: 4 -> [_]
                                n2124 = flat-sequence {
                                frame #0 {
                                n2125 = Wait (ms)(milliseconds to wait=u32 500) -> ()  [unwired: 1 out]
                                }
                                frame #1 {
                                n2126 = local read "Action (%)"() -> (w3222:dbl)
                                n2127 = Absolute Value(x=w3222) -> (abs(x)=w3221:dbl)
                                n2128 = Greater?(x=w3221, y=70.0) -> (0:w3219:bool)
                                n2129 = property on="Remove Action Offset" class="Bool (strict)"("Val(Sgnl)"=w3219) -> ()  [unwired: 2 in, 2 out]
                                }
                                }